vi "IR Opo Main.vi"() -> ()   [LabVIEW 2016] (continued)
        n224 = Close Reference(reference=w504, error in (no error)=w503) -> ()  [unwired: 1 out]
        n225 = Get Date/Time In Seconds() -> (seconds since 1Jan1904=w496:timestamp)
        n226 = Format Date/Time String(time format string (%c)="%m/%d/%y - %I:%M %p  ", seconds (now)=w496) -> (date/time string=w495:string)  [unwired: 1 in]
        n227 = Concatenate Strings(w495, "Camera started", "\r") -> (w500:string)
        n228 = invoke on="Log" class="Str" method="Append String"("string"=w500) -> (error out=w493:errorcluster)  [unwired: 3 in, 3 out]
        n229 = property on="Log" class="Str"(error in=w493, "Text.Scroll Position"=u32 500000) -> ()  [unwired: 1 in, 2 out]
        n230 = case shown="False" w525 {
          tunnel: [w530 w540] -> w514
          tunnel: w519 -> [w536 w540]
          tunnel: w517 -> [w535 w539]
          tunnel: [w535 w539] -> w516
          frame False {
            w528 = 1 items=["IS_DONT_WAIT", "IS_WAIT"] ("Wait")
            n231 = property class="Camera"(reference=w535, error in=w536) -> (error out=w537:errorcluster, "Acquisition"=w538:refnum<k24>)  [unwired: 1 out]
            n232 = invoke class="Acquisition" method="Capture"(reference=w538, error in=w537, "param"=w528) -> (reference out=w531:refnum<k24>, error out=w532:errorcluster, "Capture"=w529:i32)  [unwired: 1 in, 1 out]
            n233 = invoke class="Acquisition" method="ToString"(reference=w531, error in=w532) -> (error out=w534:errorcluster, "ToString"=w533:string)  [unwired: 1 in, 1 out]
            n234 = call "uc480_Error_Handling.vi"("Error Code"=w529, "Error String"=w533, "Error In"=w534) -> ("Error Out"=w530:errorcluster)  [unwired: 8 in]
          }
          frame True {
          }
        }
      }
    }
    n235 = call "uc480_SubVI_Example_SyncEventLoop.vi"("Error In"=w54, "use sync"=w56, ".NET (Reference)"=w55) -> ("Error Out"=w52:errorcluster, "Synchronize (ms)"=w53:dbl)  [unwired: 7 in]
    "Error Out" <- w52
    n236 = Wait Until Next ms Multiple(millisecond multiple=w53) -> ()  [unwired: 1 out]
  }
  n237 = flat-sequence "Initialization sequence" {
    tunnel: [w562] -> w8
    tunnel: [w546] -> w6
    tunnel: [w545] -> w5
    tunnel: [w542] -> w3
    tunnel: [w541] -> w2
    tunnel: w8 -> [w701]
    tunnel: [w695] -> w7
    tunnel: w6 -> [w694]
    tunnel: w5 -> [w693]
    tunnel: [w692] -> w4
    tunnel: w3 -> [w692]
    tunnel: w2 -> [w691]
    tunnel: [w691] -> w1
    tunnel: [w713] -> w19
    tunnel: [w704] -> w18
    tunnel: [w705] -> w14
    tunnel: w7 -> [w709]
    tunnel: w4 -> [w703]
    tunnel: w1 -> [w702]
    tunnel: w19 -> [w716]
    tunnel: [w716] -> w17
    tunnel: w18 -> [w715]
    tunnel: [w714] -> w15
    tunnel: w14 -> [w714]
    tunnel: w17 -> [w720]
    tunnel: [w720] -> w16
    tunnel: w15 -> [w719]
    tunnel: [w727] -> w13
    tunnel: w16 -> [w727]
    tunnel: w13 -> [w729]
    tunnel: [w729] -> w12
    tunnel: w12 -> [w731]
    tunnel: [w731] -> w11
    tunnel: w11 -> [w733]
    tunnel: [w733] -> w10
    tunnel: w10 -> [w735]
    tunnel: [w735] -> w9
    tunnel: w9 -> [w736]
    frame #0 {
      w563 = "standby" ("regular expression")
      w573 = FALSE ("Visible")
      n238 = control-ref of="This VI"() -> (w574:refnum<vi>)
      n239 = control-ref of="This VI"() -> (w572:refnum<vi>)
      n240 = invoke class="VI" method="Default Vals.Reinit All"(reference=w574) -> ()  [unwired: 2 in, 3 out]
      n241 = property on="Axes Manual Control" class="Bool (strict)"("Visible"=w573) -> ()  [unwired: 2 in, 2 out]
      n242 = property on="Home Axes" class="Bool"("Visible"=w573) -> ()  [unwired: 2 in, 2 out]
      n243 = property class="VI"(reference=w572) -> ("Path"=w571:path)  [unwired: 1 in, 2 out]
      n244 = Strip Path(path=w571) -> (stripped path=w570:path)  [unwired: 1 out]
      n245 = Build Path(base path=w570, name or relative path="General_Configuration.ini") -> (appended path=w568:path)
      n246 = call <vilib>:"Open Config Data.vi"("create file if necessary (T)"=FALSE, "configuration file path"=w568) -> ("error out"=w543:errorcluster, "refnum"=w544:T5)  [unwired: 7 in, 1 out]
      n247 = call "Configuration reader.vi"("refnum"=w544, "error in (no error)"=w543) -> ("Velocity"=→"Velocity":dbl, "X offset"=w555:i32, "Y travel"=w553:dbl, "X travel"=w552:dbl, "Y offset"=w554:i32, "Acceleration"=→"Acceleration":dbl, "Width (px)"=w557:i32, "Speed (µm/s)"=w561:i32, "XPS_Address"=→"XPS_Address":string, "Axis 1 group"=w542:i32, "Precision (%)"=w558:dbl, "Pixel size"=w559:dbl, "Heigth (px)"=w556:i32, "Laser Com Delay"=w545:i32, "Height  step \ndivider"=w560:i32, "VISA Laser port"=w546:string, "Axis 2 group"=w541:i32, "error out"=w548:errorcluster)
      "VISA Laser port" <- w546
      "Laser Com Delay" <- w545
      "Axis 1 group" <- w542
      "Axis 2 group" <- w541
      n248 = local write "Height  step \ndivider"(w560) -> ()
      n249 = local write "Heigth (px)"(w556) -> ()
      n250 = local write "Pixel size"(w559) -> ()
      n251 = local write "Precision (%)"(w558) -> ()
      n252 = local write "Speed (µm/s)"(w561) -> ()
      n253 = local write "Width (px)"(w557) -> ()
      n254 = local write "X offset"(w555) -> ()
      n255 = local write "X travel"(w552) -> ()
      n256 = local write "Y offset"(w554) -> ()
      n257 = local write "Y travel"(w553) -> ()
      n258 = call "CheckStatus.vi"("Error In"=w548, "delay before read (ms)"=w545, "VISA resource name"=w546) -> ("Error Out"=w547:errorcluster, "read buffer"=w566:string)  [unwired: 5 in, 2 out]
      n259 = xnode "Match Regular Expression"("input string"=w566, "regular expression"=w563, "error in"=w547) -> ("whole match"=w564:string, "error out"=w562:errorcluster)  [unwired: 3 in, 3 out]
      n260 = Equal?(x=w564, y=w563) -> (x = y?=w565:bool)
      n261 = case shown="True" w565 {
        frame False {
        }
        frame True {
          n262 = control-ref of="Log"() -> (w690:refnum<vi>)
          n263 = call "Log writer.vi"("reference"=w690, "string"="Initializing the ICE450 Ultra..." ("Initialiazation")) -> ()  [unwired: 10 in]
        }
      }
    }
    frame #1 {
      n264 = call "ICE450 Ultra Initialization.vi"("error in (no error)"=w701, "delay before read (ms)"=w693, "VISA resource name"=w694) -> ("Error Out"=w695:errorcluster, "Repetition rate"=w696:dbl, "Laser initialization status"=w700:string)  [unwired: 6 in]
      n265 = local write "Repetition\nRate (Hz)"(w696) -> ()
      n266 = property on="Log" class="Str"("Text.Scroll Position"=u32 500000) -> ()  [unwired: 2 in, 2 out]
      n267 = Concatenate Strings(w700, "\r") -> (w698:string)
      n268 = invoke on="Log" class="Str" method="Append String"("string"=w698) -> ()  [unwired: 3 in, 4 out]
    }
    frame #2 {
      n269 = local read "XPS_Address"() -> (w706:string)
      n270 = control-ref of="Log"() -> (w707:refnum<vi>)
      n271 = call "Axes initialization.vi"("Axis 2 group"=w702, "Axis 1 group"=w703, "error in (no error)"=w709, "Axis Initial Parameters"="Axis Initial Parameters", "reference"=w707, "XPS_Address"=w706) -> ("Error out"=w710:errorcluster, "Axis 1"=→"Axis 1":string, "Axis 1 ready?"=w704:bool, "Axis 2"=→"Axis 2":string, "Axes 2 ready?"=w705:bool)
      n272 = call <vilib>:"Simple Error Handler.vi"("error in (no error)"=w710) -> ()  [unwired: 4 in, 5 out]
      n273 = And(x=w704, y=w705) -> (x .and. y?=w713:bool)
    }
    frame #3 {
      n274 = case shown="True" w715 {
        frame False {
        }
        frame True {
          n275 = control-ref of="Log"() -> (w718:refnum<vi>)
          n276 = call "Log writer.vi"("reference"=w718, "string"="Axis 1 ready" ("Initialiazation")) -> ()  [unwired: 10 in]
        }
      }
    }
    frame #4 {
      n277 = case shown="True" w719 {
        frame False {
        }
        frame True {
          n278 = control-ref of="Log"() -> (w721:refnum<vi>)
          n279 = call "Log writer.vi"("reference"=w721, "string"="Axis 2 ready" ("Initialiazation")) -> ()  [unwired: 10 in]
        }
      }
    }
    frame #5 {
      w723 = FALSE ("Visible")
      # "Set defaults"
      n280 = property on="LAMP" class="Bool (strict)"("BoolText.Text"="LAMP OFF" ("Boolean Text.Text")) -> ()  [unwired: 2 in, 2 out]
      n281 = property on="Laser Operation" class="Bool (strict)"("Blinking"=w723) -> ()  [unwired: 2 in, 2 out]
      n282 = property on="Capture" class="Bool"("Visible"=w723) -> ()  [unwired: 2 in, 2 out]
      n283 = property on="SINGLE SHOT" class="Bool"("Visible"=w723) -> ()  [unwired: 2 in, 2 out]
      n284 = property on="LASER" class="Bool (strict)"("BoolText.Text"="LASER OFF" ("Boolean Text.Text"), "Visible"=FALSE) -> ()  [unwired: 2 in, 2 out]
    }
    frame #6 {
      n285 = local write "Camera Status"("Init camera" ("Camera Status")) -> ()
    }
    frame #7 {
      n286 = Wait (ms)(milliseconds to wait=u32 1000) -> ()  [unwired: 1 out]
    }
    frame #8 {
      n287 = local write "Camera Status"("Start live") -> ()
    }
    frame #9 {
      n288 = Wait (ms)(milliseconds to wait=u32 1000) -> ()  [unwired: 1 out]
    }
    frame #10 {
      n289 = case shown="True" w736 {
        frame False {
          n290 = One Button Dialog(message="Axes not ready") -> ()  [unwired: 1 in, 1 out]
        }
        frame True {
          n291 = property on="Axes Manual Control" class="Bool (strict)"("Visible"=TRUE) -> ()  [unwired: 2 in, 2 out]
          n292 = property on="Home Axes" class="Bool"("Visible"=TRUE) -> ()  [unwired: 2 in, 2 out]
          n293 = control-ref of="Log"() -> (w739:refnum<vi>)
          n294 = call "Log writer.vi"("reference"=w739, "string"="System ready" ("Initialiazation")) -> ()  [unwired: 10 in]
        }
      }
    }
  }
  n295 = while "Laser control & Stages Control" {
    stop <- w754 stop-if-true
    n296 = local read "Laser Com Delay"() -> (w742:i32)
    n297 = local read "VISA Laser port"() -> (w743:string)
    n298 = local read "XPS_Address"() -> (w746:string)
    n299 = local read "Axis 2"() -> (w744:string)
    n300 = local read "Axis 1"() -> (w745:string)
    n301 = event shown="[11] \"Process Image\": Value Change" {
      selector: _ -> [_ _ _ _ _ _ _ _ _ _ _ _ _ _ _ _ _ _ _ _]
      dyn-events: _ -> [_ _ _ _ _ _ _ _ _ _ _ _ _ _ _ _ _ _ _ _]
      timeout: _ -> [_ _ _ _ _ _ _ _ _ _ _ _ _ _ _ _ _ _ _ _]
      tunnel: [_ _ _ w1086 _ _ _ _ _ _ _ _ _ _ _ _ _ _ _ _] -> w754
      tunnel: [w761 w917 w1080 _ _ _ w1141 _ w1169 w1196 _ w1257 _ _ _ "" ("StringOut") w1516 _ w1640 w1743] -> w747
      tunnel: w746 -> [_ _ _ _ _ _ _ _ _ w1199 _ _ _ _ _ w1435 w1515 _ w1627 w1732]
      tunnel: w745 -> [_ _ _ _ _ _ _ _ _ w1198 _ _ _ _ _ w1434 w1514 _ w1626 w1744]
      tunnel: w744 -> [_ _ _ _ _ _ _ _ _ w1197 _ _ _ _ _ w1433 w1513 _ w1625 w1745]
      tunnel: w743 -> [w759 w915 w1077 w1085 _ _ w1144 w1164 _ _ _ _ _ _ _ _ _ _ _ _]
      tunnel: w742 -> [w758 w914 w1076 w1084 _ _ w1143 w1163 _ _ _ _ _ _ _ _ _ _ _ _]
      event "LAMP": Value Change {
        n302 = event-data() -> ()  [unwired: 1 in, 6 out]
        n303 = case shown="True" "LAMP" {
          tunnel: [w762 w890] -> w761
          tunnel: w759 -> [w768 w889]
          tunnel: w758 -> [w767 w888]
          frame False {
            w763 = "standby" ("regular expression")
            n304 = call "FLStop.vi"("delay before read (ms)"=w767, "VISA resource name"=w768) -> ("read buffer"=w766:string)  [unwired: 6 in, 3 out]
            n305 = xnode "Match Regular Expression"("input string"=w766, "regular expression"=w763) -> ("whole match"=w764:string)  [unwired: 4 in, 4 out]
            n306 = Equal?(x=w764, y=w763) -> (x = y?=w765:bool)
            n307 = case shown="True" w765 {
              tunnel: ["" "Flashlamp deactivated"] -> w762
              frame False {
              }
              frame True {
                w770 = FALSE ("Visible")
                n308 = property on="LASER" class="Bool (strict)"("Visible"=w770) -> ()  [unwired: 2 in, 2 out]
                n309 = property on="Capture" class="Bool"("Visible"=w770) -> ()  [unwired: 2 in, 2 out]
                n310 = property on="SINGLE SHOT" class="Bool"("Visible"=w770) -> ()  [unwired: 2 in, 2 out]
                n311 = property on="Laser Operation" class="Bool (strict)"("Blinking"=w770) -> ()  [unwired: 2 in, 2 out]
                n312 = property on="LAMP" class="Bool (strict)"("BoolText.Text"="LAMP OFF" ("Boolean Text.Text")) -> ()  [unwired: 2 in, 2 out]
              }
            }
          }
          frame True {
            n313 = flat-sequence {
              tunnel: w889 -> [w898]
              tunnel: w888 -> [w897]
              tunnel: [w894] -> w887
              tunnel: [w908] -> w890
              tunnel: w887 -> [w907]
              frame #0 {
                w895 = "fire" ("regular expression")
                n314 = while {
                  i -> [w902]
                  stop <- w905 stop-if-true
                  n315 = Wait Until Next ms Multiple(millisecond multiple=u32 1000) -> ()  [unwired: 1 out]
                  n316 = Equal?(x=5, y=w902) -> (x = y?=w905:bool)
                  n317 = Subtract(x=5, y=w902) -> (x-y=w900:i32)
                  n318 = Number To Decimal String(number=w900) -> (decimal integer string=w901:string)  [unwired: 1 in]
                  n319 = property on="LAMP" class="Bool (strict)"("BoolText.Text"=w901) -> ()  [unwired: 2 in, 2 out]
                }
                n320 = Wait (ms)(milliseconds to wait=u32 5000) -> ()  [unwired: 1 out]
                n321 = call "FLStart.vi"("delay before read (ms)"=w897, "VISA resource name"=w898) -> ("Error Out"=w892:errorcluster, "read buffer"=w893:string)  [unwired: 6 in, 2 out]
                n322 = Match Pattern(string=w893, regular expression=w895) -> (match substring=w896:string)  [unwired: 1 in, 3 out]
                n323 = call <vilib>:"Simple Error Handler.vi"("error source (\" \")"="Lamp" ("error source (\" \")"), "error in (no error)"=w892) -> ()  [unwired: 3 in, 5 out]
                n324 = Equal?(x=w896, y=w895) -> (x = y?=w894:bool)
              }
              frame #1 {
                n325 = case shown="True" w907 {
                  tunnel: ["Flashlamp NOT firing" "Flashlamp activated"] -> w908
                  frame False {
                    n326 = property on="LAMP" class="Bool (strict)"("Value"=FALSE ("LAMP")) -> ()  [unwired: 2 in, 2 out]
                  }
                  frame True {
                    w911 = TRUE ("Visible")
                    n327 = property on="LASER" class="Bool (strict)"("Visible"=w911) -> ()  [unwired: 2 in, 2 out]
                    n328 = property on="Capture" class="Bool"("Visible"=w911) -> ()  [unwired: 2 in, 2 out]
                    n329 = property on="LAMP" class="Bool (strict)"("BoolText.Text"="LAMP ON" ("Boolean Text.Text")) -> ()  [unwired: 2 in, 2 out]
                    n330 = property on="SINGLE SHOT" class="Bool"("Visible"=w911) -> ()  [unwired: 2 in, 2 out]
                  }
                }
              }
            }
          }
        }
      }
      event "LASER": Value Change {
        n331 = event-data() -> ()  [unwired: 1 in, 6 out]
        n332 = case shown="False" "LASER" {
          tunnel: [w928 w1057] -> w918
          tunnel: [w927 w1056] -> w917
          tunnel: w915 -> [w925 w1051]
          tunnel: w914 -> [w924 w1050]
          frame False {
            w922 = "fire" ("regular expression")
            n333 = local read "LAMP"() -> (w926:bool)
            n334 = case shown="True" w926 {
              tunnel: [FALSE ("Visible") TRUE ("Visible")] -> w919
              frame False {
              }
              frame True {
              }
            }
            n335 = property on="Capture" class="Bool"("Visible"=w919) -> ()  [unwired: 2 in, 2 out]
            n336 = property on="SINGLE SHOT" class="Bool"("Visible"=w919) -> ()  [unwired: 2 in, 2 out]
            n337 = call "QSStop.vi"("delay before read (ms)"=w924, "VISA resource name"=w925) -> ("read buffer"=w921:string)  [unwired: 6 in, 3 out]
            n338 = xnode "Match Regular Expression"("input string"=w921, "regular expression"=w922) -> ("whole match"=w923:string)  [unwired: 4 in, 4 out]
            n339 = Equal?(x=w923, y=w922) -> (x = y?=w920:bool)
            n340 = case shown="False" w920 {
              tunnel: [FALSE w932] -> w928
              tunnel: ["" "Q-Switch deactivated"] -> w927
              frame False {
              }
              frame True {
                w932 = FALSE ("Boolean")
                n341 = property on="LASER" class="Bool (strict)"("BoolText.Text"="LASER OFF" ("Boolean Text.Text"), "Value"=w932) -> ()  [unwired: 2 in, 2 out]
                n342 = property on="Laser Operation" class="Bool (strict)"("Blinking"=w932) -> ()  [unwired: 2 in, 2 out]
              }
            }
          }
          frame True {
            w1053 = "fire" ("regular expression")
            n343 = call "CheckStatus.vi"("delay before read (ms)"=w1050, "VISA resource name"=w1051) -> ("read buffer"=w1055:string)  [unwired: 6 in, 3 out]
            n344 = Match Pattern(string=w1055, regular expression=w1053) -> (match substring=w1054:string)  [unwired: 1 in, 3 out]
            n345 = Equal?(x=w1054, y=w1053) -> (x = y?=w1052:bool)
            n346 = case shown="True" w1052 {
              tunnel: [FALSE ("Boolean") w1068] -> w1057
              tunnel: ["The flashlamp is not firing" w1067] -> w1056
              tunnel: w1051 -> [_ w1066]
              tunnel: w1050 -> [_ w1065]
              frame False {
                n347 = property on="LASER" class="Bool (strict)"("Value"=FALSE ("LASER")) -> ()  [unwired: 2 in, 2 out]
              }
              frame True {
                w1063 = "qs" ("regular expression")
                n348 = call "QSStart.vi"("delay before read (ms)"=w1065, "VISA resource name"=w1066) -> ("read buffer"=w1062:string)  [unwired: 6 in, 3 out]
                n349 = Match Pattern(string=w1062, regular expression=w1063) -> (match substring=w1064:string)  [unwired: 1 in, 3 out]
                n350 = Equal?(x=w1064, y=w1063) -> (x = y?=w1061:bool)
                n351 = case shown="True" w1061 {
                  tunnel: [FALSE ("Boolean") w1074] -> w1068
                  tunnel: ["Q-Switch is NOT firing" "Q-Switch activated"] -> w1067
                  frame False {
                    n352 = property on="LASER" class="Bool (strict)"("Value"=FALSE ("LASER")) -> ()  [unwired: 2 in, 2 out]
                  }
                  frame True {
                    w1072 = FALSE ("Visible")
                    w1074 = TRUE ("Boolean")
                    n353 = property on="Capture" class="Bool"("Visible"=w1072) -> ()  [unwired: 2 in, 2 out]
                    n354 = property on="Laser Operation" class="Bool (strict)"("Blinking"=w1074) -> ()  [unwired: 2 in, 2 out]
                    n355 = property on="LASER" class="Bool (strict)"("BoolText.Text"="LASER ON" ("Boolean Text.Text")) -> ()  [unwired: 2 in, 2 out]
                    n356 = property on="SINGLE SHOT" class="Bool"("Visible"=w1072) -> ()  [unwired: 2 in, 2 out]
                  }
                }
              }
            }
          }
        }
        "Laser Operation" <- w918
      }
      event "Repetition\nRate (Hz)": Value Change {
        n357 = event-data() -> ()  [unwired: 1 in, 6 out]
        n358 = call "FLFrequencySet.vi"("Frequency (Hz)"="Repetition\nRate (Hz)", "delay before read (ms)"=w1076, "VISA resource name"=w1077) -> ()  [unwired: 5 in, 4 out]
        n359 = Number To Fractional String(number="Repetition\nRate (Hz)", precision (6)=i16 2 ("width (-)")) -> (F-format string=w1082:string)  [unwired: 2 in]
        n360 = Concatenate Strings("Repetition rate set to: " ("string"), w1082, " Hz" ("string")) -> (w1080:string)
      }
      event "EXIT": Value Change {
        n361 = event-data() -> ()  [unwired: 1 in, 6 out]
        n362 = flat-sequence {
          tunnel: w1085 -> [w1088]
          tunnel: w1084 -> [w1087]
          tunnel: ["EXIT"] -> w1086
          frame #0 {
            n363 = call "QSStop.vi"("delay before read (ms)"=w1087, "VISA resource name"=w1088) -> ("Error Out"=w1089:errorcluster)  [unwired: 6 in, 3 out]
            n364 = call "FLStop.vi"("Error In"=w1089, "delay before read (ms)"=w1087, "VISA resource name"=w1088) -> ()  [unwired: 5 in, 4 out]
          }
          frame #1 {
            n365 = Wait (ms)(milliseconds to wait=u32 1000) -> ()  [unwired: 1 out]
          }
          frame #2 {
            n366 = local write "Camera Status"("Exit camera") -> ()
          }
          frame #3 {
            n367 = Wait (ms)(milliseconds to wait=u32 1000) -> ()  [unwired: 1 out]
          }
          frame #4 {
            n368 = control-ref of="This Application"() -> (w1112:refnum<vi>)
            n369 = control-ref of="This VI"() -> (w1096:refnum<vi>)
            n370 = property class="VI"(reference=w1096) -> ("Path"=w1097:path)  [unwired: 1 in, 2 out]
            n371 = property class="App"(reference=w1112) -> ("App.Kind"=w1111:T8)  [unwired: 1 in, 2 out]
            n372 = Strip Path(path=w1097) -> (stripped path=w1106:path)  [unwired: 1 out]
            n373 = case shown="\"Run Time System\"" w1111 {
              frame "Development System", Default {
              }
              frame "Run Time System" {
                n374 = control-ref of="This VI"() -> (w1121:refnum<vi>)
                n375 = invoke class="VI" method="FP.Close"(reference=w1121) -> ()  [unwired: 2 in, 3 out]
                n376 = Quit LabVIEW() -> ()  [unwired: 1 in]
              }
            }
            n377 = Build Path(base path=w1106, name or relative path="Logs") -> (appended path=w1104:path)
            n378 = call <vilib>:"Check if File or Folder Exists.vi"("path"=w1104) -> ("file or folder exists?"=w1105:bool, "dup path"=w1107:path)  [unwired: 8 in, 1 out]
            n379 = case shown="False" w1105 {
              tunnel: w1107 -> [w1114 w1115]
              tunnel: [w1113 w1115] -> w1110
              frame False {
                n380 = Create Folder(path (use dialog)=w1114) -> (created path=w1113:path)  [unwired: 2 in, 2 out]
              }
              frame True {
              }
            }
            n381 = Get Date/Time In Seconds() -> (seconds since 1Jan1904=w1101:timestamp)
            n382 = Format Date/Time String(time format string (%c)="%d%m%y %I-%M %p ", seconds (now)=w1101) -> (date/time string=w1099:string)  [unwired: 1 in]
            n383 = Concatenate Strings(w1099, "Log File.txt") -> (w1109:string)
            n384 = Build Path(base path=w1110, name or relative path=w1109) -> (appended path=w1108:path)
            n385 = Open/Create/Replace File(file path (use dialog)=w1108, operation (0:open)=T6."replace or create") -> (refnum out=w1095:refnum<file>, cancelled=w1093:bool, error out=w1094:errorcluster)  [unwired: 4 in]
            n386 = case shown="False" w1093 {
              tunnel: w1095 -> [w1120 _]
              tunnel: w1094 -> [w1118 _]
              frame False {
                n387 = local read "Log"() -> (w1119:string)
                n388 = Write to Text File(file (use dialog)=w1120, text=w1119, error in=w1118) -> (refnum out=w1117:refnum<file>, error out=w1116:errorcluster)  [unwired: 2 out]
                n389 = Close File(refnum=w1117, error in=w1116) -> ()  [unwired: 2 out]
              }
              frame True {
              }
            }
          }
          frame #5 {
          }
        }
      }
      event "Processing time unit", "Processi time (sec)": Value Change {
        n390 = event-data() -> ()  [unwired: 1 in, 6 out]
        n391 = local read "Processing time unit"() -> (w1125:string)
        n392 = Equal?(x=w1125, y="min") -> (x = y?=w1123:bool)
        n393 = case shown="False" w1123 {
          frame False {
            n394 = local read "Processi time (sec)"() -> (w1126:i32)
            n395 = local write "Process time"(w1126) -> ()
          }
          frame True {
            n396 = local read "Processi time (sec)"() -> (w1128:i32)
            n397 = Quotient & Remainder(x=w1128, y=60) -> (floor(x/y)=w1127:i32)  [unwired: 1 out]
            n398 = local write "Process time"(w1127) -> ()
          }
        }
      }
      event "Overlay MSI Image": Value Change {
        n399 = event-data() -> ()  [unwired: 1 in, 6 out]
        n400 = vi-ref "MSI_Image_overlap.vi"() -> (w1130:refnum<vi>)
        n401 = case shown="True" "Overlay MSI Image" {
          tunnel: w1130 -> [_ w1135]
          frame False {
          }
          frame True {
            n402 = invoke class="VI" method="FP.Open"(reference=w1135, "Activate"=TRUE ("Activate?"), "State"=T7."Standard") -> (reference out=w1138:refnum<vi>, error out=w1133:errorcluster)  [unwired: 2 in, 3 out]
            n403 = invoke class="VI" method="Run VI"(reference=w1138, error in=w1133, "Wait until done"=FALSE ("Wait Until Done"), "Auto Dispose Ref"=TRUE ("Auto Dispose Reference")) -> (reference out=w1134:refnum<vi>, error out=w1132:errorcluster)  [unwired: 1 in, 3 out]
            n404 = Close Reference(reference=w1134, error in (no error)=w1132) -> ()  [unwired: 1 out]
          }
        }
      }
      event "SINGLE SHOT": Value Change {
        n405 = event-data() -> ()  [unwired: 1 in, 6 out]
        n406 = case shown="True" "SINGLE SHOT" {
          tunnel: w1144 -> [_ w1148]
          tunnel: w1143 -> [_ w1147]
          tunnel: ["" w1146] -> w1141
          frame False {
          }
          frame True {
            w1152 = "fire" ("regular expression")
            n407 = call "CheckStatus.vi"("delay before read (ms)"=w1147, "VISA resource name"=w1148) -> ("read buffer"=w1150:string)  [unwired: 6 in, 3 out]
            n408 = Match Pattern(string=w1150, regular expression=w1152) -> (match substring=w1151:string)  [unwired: 1 in, 3 out]
            n409 = Equal?(x=w1151, y=w1152) -> (x = y?=w1149:bool)
            n410 = case shown="True" w1149 {
              tunnel: ["The flashlamp is not firing" w1160] -> w1146
              tunnel: w1148 -> [_ w1159]
              tunnel: w1147 -> [_ w1158]
              frame False {
              }
              frame True {
                w1156 = "qs" ("regular expression")
                n411 = call "QSSingleShot.vi"("delay before read (ms)"=w1158, "VISA resource name"=w1159) -> ("read buffer"=w1155:string)  [unwired: 6 in, 3 out]
                n412 = Match Pattern(string=w1155, regular expression=w1156) -> (match substring=w1157:string)  [unwired: 1 in, 3 out]
                n413 = Equal?(x=w1157, y=w1156) -> (x = y?=w1154:bool)
                n414 = case shown="True" w1154 {
                  tunnel: ["Q-Switch is NOT firing" "Q-Switch activated"] -> w1160
                  frame False {
                  }
                  frame True {
                  }
                }
              }
            }
          }
        }
      }
      event "Laser Status": Value Change {
        n415 = event-data() -> ()  [unwired: 1 in, 6 out]
        n416 = case shown="True" "Laser Status" {
          tunnel: w1164 -> [_ w1167]
          tunnel: w1163 -> [_ w1166]
          frame False {
          }
          frame True {
            n417 = call "ICE450UltraMonitor.vi"("delay before read (ms)"=w1166, "VISA resource name"=w1167) -> ()  [unwired: 10 in]
          }
        }
      }
      event "Open \nManual": Value Change {
        n418 = event-data() -> ()  [unwired: 1 in, 6 out]
        n419 = case shown="True" "Open \nManual" {
          tunnel: [_ "Opening Manual" ("StringOut")] -> w1169
          frame False {
          }
          frame True {
            w1178 = FALSE  # wait until completion? (T)
            n420 = control-ref of="This VI"() -> (w1182:refnum<vi>)
            n421 = property class="VI"(reference=w1182) -> ("Path"=w1181:path)  [unwired: 1 in, 2 out]
            n422 = Strip Path(path=w1181) -> (stripped path=w1180:path)  [unwired: 1 out]
            n423 = Build Path(base path=w1180, name or relative path="LAST_Software_Manual.PDF") -> (appended path=w1172:path)
            n424 = Path To String(path=w1172) -> (string=w1175:string)
            n425 = Concatenate Strings("cmd  /c \"", w1175, "\"" ("string")) -> (w1170:string)
            n426 = call <vilib>:"System Exec.vi"("run minimized? (F)"=TRUE, "wait until completion? (T)"=w1178, "error in (no error)"="error in (no error)", "command line"=w1170) -> ("error out"=→"error out":errorcluster)  [unwired: 4 in, 3 out]
          }
        }
      }
      event "Stages status": Value Change {
        w1190 = "Ready"
        n427 = event-data() -> ()  [unwired: 1 in, 6 out]
        n428 = case shown="True" "Stages status" {
          tunnel: w1199 -> [_ w1212]
          tunnel: w1198 -> [_ w1211]
          tunnel: w1197 -> [_ w1210]
          tunnel: [w1203 w1209] -> w1196
          tunnel: [w1203 w1207] -> w1186
          tunnel: [w1203 w1208] -> w1185
          frame False {
            w1203 = ""
          }
          frame True {
            n429 = call <userlib>:"Open TCP-IP.vi"("IP address"=w1212) -> ("error out"=w1206:errorcluster, "Connection ID"=w1213:T9)  [unwired: 8 in, 1 out]
            n430 = call <vilib>:"Simple Error Handler.vi"("error in (no error)"=w1206) -> ("error?"=w1204:bool, "error out"=w1205:errorcluster)  [unwired: 4 in, 3 out]
            n431 = case shown="False" w1204 {
              tunnel: w1213 -> [w1234 _]
              tunnel: w1205 -> [w1233 _]
              tunnel: w1211 -> [w1226 _]
              tunnel: w1210 -> [w1225 _]
              tunnel: [w1224 w1235] -> w1209
              tunnel: [w1221 w1235] -> w1208
              tunnel: [w1217 w1235] -> w1207
              frame False {
                n432 = call "Get Stages Status.vi"("error in (no error)"=w1233, "Group Name (250 c max)"=w1226, "connection ID in"=w1234) -> ("error out"=w1230:errorcluster, "XPS error out"=w1229:errorcluster, "Group Status String"=w1221:string, "connection ID out"=w1232:T9)  [unwired: 4 in, 1 out]
                n433 = call "Get Stages Status.vi"("error in (no error)"=w1230, "XPS error in (no error)"=w1229, "Group Name (250 c max)"=w1225, "connection ID in"=w1232) -> ("error out"=w1227:errorcluster, "XPS error out"=w1223:errorcluster, "Group Status String"=w1217:string, "connection ID out"=w1228:T9)  [unwired: 3 in, 1 out]
                n434 = call <vilib>:"Simple Error Handler.vi"("error source (\" \")"="Stage status" ("error source (\" \")"), "error in (no error)"=w1223) -> ()  [unwired: 3 in, 5 out]
                n435 = Concatenate Strings("Axis 1 " ("string"), w1221) -> (w1220:string)
                n436 = call <userlib>:"Close TCP-IP.vi"("error in (no error)"=w1227, "connection ID in"=w1228) -> ("Error out"=w1222:errorcluster)  [unwired: 9 in]
                n437 = call <vilib>:"Simple Error Handler.vi"("error source (\" \")"="TCP close Stage status" ("error source (\" \")"), "error in (no error)"=w1222) -> ()  [unwired: 3 in, 5 out]
                n438 = Concatenate Strings("Axis 2 " ("string"), w1217) -> (w1218:string)
                n439 = Concatenate Strings(w1220, " - " ("string"), w1218) -> (w1224:string)
              }
              frame True {
                w1235 = ""
              }
            }
          }
        }
        n440 = String Subset(string=w1185, offset (0)=0, length (rest)=5 ("length (rest)")) -> (substring=w1189:string)
        n441 = String Subset(string=w1186, offset (0)=0, length (rest)=5 ("length (rest)")) -> (substring=w1191:string)
        n442 = Equal?(x=w1190, y=w1189) -> (x = y?=w1187:bool)
        n443 = Equal?(x=w1191, y=w1190) -> (x = y?=w1188:bool)
        n444 = And(x=w1188, y=w1187) -> (x .and. y?=w1184:bool)
        n445 = case shown="True" w1184 {
          frame False {
          }
          frame True {
            n446 = property on="Axes Manual Control" class="Bool (strict)"("Visible"=TRUE) -> ()  [unwired: 2 in, 2 out]
            n447 = property on="Home Axes" class="Bool"("Visible"=TRUE) -> ()  [unwired: 2 in, 2 out]
          }
        }
      }
      event "Save configuration": Value Change {
        n448 = event-data() -> ()  [unwired: 1 in, 6 out]
        n449 = case shown="True" "Save configuration" {
          frame False {
          }
          frame True {
            n450 = control-ref of="This VI"() -> (w1255:refnum<vi>)
            n451 = property class="VI"(reference=w1255) -> ("Path"=w1254:path)  [unwired: 1 in, 2 out]
            n452 = Strip Path(path=w1254) -> (stripped path=w1253:path)  [unwired: 1 out]
            n453 = local read "Height  step \ndivider"() -> (w1248:i32)
            n454 = Build Path(base path=w1253, name or relative path="General_Configuration.ini") -> (appended path=w1251:path)
            n455 = local read "Speed (µm/s)"() -> (w1244:i32)
            n456 = local read "Precision (%)"() -> (w1245:dbl)
            n457 = local read "Heigth (px)"() -> (w1247:i32)
            n458 = local read "Width (px)"() -> (w1243:i32)
            n459 = local read "Pixel size"() -> (w1246:dbl)
            n460 = local read "X offset"() -> (w1242:i32)
            n461 = local read "X travel"() -> (w1240:dbl)
            n462 = local read "Y offset"() -> (w1241:i32)
            n463 = local read "Y travel"() -> (w1239:dbl)
            n464 = call <vilib>:"Open Config Data.vi"("create file if necessary (T)"=FALSE, "configuration file path"=w1251) -> ("error out"=w1238:errorcluster, "refnum"=w1249:T5)  [unwired: 7 in, 1 out]
            n465 = call "Configuration writer.vi"("Path"=w1249, "Width (px)"=w1243, "error in (no error)"=w1238, "Precision (%)"=w1245, "Heigth (px)"=w1247, "X offset"=w1242, "X travel"=w1240, "Y offset"=w1241, "Speed (µm/s)"=w1244, "Height  step \ndivider"=w1248, "Y travel"=w1239, "Pixel size"=w1246) -> ("error out"=w1237:errorcluster)  [unwired: 7 in]
            n466 = call <vilib>:"Simple Error Handler.vi"("error in (no error)"=w1237) -> ()  [unwired: 4 in, 5 out]
          }
        }
      }
      event "Process Image": Value Change {
        n467 = event-data() -> ()  [unwired: 1 in, 6 out]
        n468 = case shown="True" "Process Image" {
          tunnel: ["" "Processing done"] -> w1257
          frame False {
          }
          frame True {
            (unwired) "untitled" ("Image Name")
            w1291 = 2 ("y")
            w1318 = 0.5  # Delay after laser on/off
            w1352 = T10 0 items=["Grayscale (U8)", "Grayscale (I16)", "Grayscale (SGL)", "Complex (CSG)", "RGB (U32)", "HSL (U32)", "RGB (U64)", "Grayscale (U16)"] ("Image Type")
            w1355 = i16 4 ("precision (6)")
            w1349 = 1000 ("y")
            n469 = control-ref of="This VI"() -> (w1263:refnum<vi>)
            n470 = control-ref of="This VI"() -> (w1271:refnum<vi>)
            n471 = local read "Source"() -> (w1354:T2)
            n472 = call "IMAQ Create"("Image Name"="untitled") -> ("New Image"=w1260:T2)  [unwired: 4 in, 1 out]
            n473 = property class="VI"(reference=w1263) -> ("Path"=w1264:path)  [unwired: 1 in, 2 out]
            n474 = property class="VI"(reference=w1271) -> ("Path"=w1270:path)  [unwired: 1 in, 2 out]
            n475 = property on="Source" class="ImageControl"() -> ("ROI"=w1261:T11)  [unwired: 2 in, 2 out]
            n476 = call "IMAQ ROIToMask 2"("ROI Descriptor"=w1261, "Image"=w1260) -> ("Image Out"=w1259:T2)  [unwired: 7 in, 2 out]
            n477 = call "IMAQ Cast Image"("Image Type"=w1352, "Image Src"=w1354) -> ("error out"=w1303:errorcluster, "Image Dst Out"=w1353:T2)  [unwired: 8 in]
            n478 = Unbundle By Name(w1261) -> ("Global Rectangle"=w1308:i32[])
            n479 = Strip Path(path=w1264) -> (stripped path=w1265:path)  [unwired: 1 out]
            n480 = Strip Path(path=w1270) -> (stripped path=w1269:path)  [unwired: 1 out]
            n481 = call "IMAQ ROIToMask 2"("error in (no error)"=w1303, "ROI Descriptor"=w1261, "Image"=w1353) -> ("error out"=w1304:errorcluster, "Image Out"=w1356:T2)  [unwired: 6 in, 1 out]
            n482 = Build Path(base path=w1265, name or relative path="Last_ROI.TIFF") -> (appended path=w1267:path)
            n483 = call-poly "IMAQ Write File 2"("File Path"=w1267, "Image"=w1259) -> ()  [unwired: 8 in, 2 out]
            n484 = Build Path(base path=w1269, name or relative path="Last_ROI.TIFF") -> ()  [unwired: 1 out]
            n485 = call "IMAQ ImageToArray"("error in (no error)"=w1304, "Image"=w1356) -> ("error out"=w1302:errorcluster, "Image Pixels (U8)"=w1274:u8[][])  [unwired: 2 in, 3 out]
            n486 = Array To Cluster(array=w1308) -> (cluster=w1307:T12)
            n487 = local read "Y offset"() -> (w1283:i32)
            n488 = local read "X offset"() -> (w1284:i32)
            n489 = call <vilib>:"Simple Error Handler.vi"("error in (no error)"=w1302) -> ()  [unwired: 4 in, 5 out]
            n490 = Unbundle(w1307) -> ("Global Rectangle[0]"=w1306:i32, "Global Rectangle[1]"=w1305:i32)
            n491 = Subtract(x=w1306, y=w1283) -> (x-y=w1297:i32)
            n492 = Subtract(x=w1305, y=w1284) -> (x-y=w1288:i32)
            n493 = local read "Width (px)"() -> (w1272:i32)
            n494 = call "ROI corrector.vi"("ROI"=w1274, "Spot diameter"=w1272) -> ("Corrected ROI"=w1273:u8[][])  [unwired: 9 in]
            n495 = Empty Array?(array=w1273) -> (empty?=w1340:bool)
            n496 = case shown="False" w1340 {
              tunnel: [w1363 u8[][] [[1]] ("Image Pixels (U8)")] -> w1339
              tunnel: w1273 -> [w1363 _]
              frame False {
              }
              frame True {
                n497 = One Button Dialog(message="ATTENTION: you did not select\nany region of interest") -> ()  [unwired: 1 in, 1 out]
              }
            }
            n498 = local read "Heigth (px)"() -> (w1290:i32)
            n499 = Divide(x=w1272, y=2.0) -> (x/y=w1279:dbl)
            n500 = Divide "Spot height radius"(x=w1290, y=w1291) -> (x/y=w1292:dbl)
            n501 = Divide "Spot width radius"(x=w1272, y=w1291) -> (x/y=w1295:dbl)
            n502 = Initialize Array(1 ("element"), w1272, w1272) -> (w1280:i32[][])
            n503 = Round To Nearest(number=w1279) -> (nearest integer value=w1277:dbl)
            n504 = call "circle spot calculator.vi"("Center Y"=w1277, "Radius"=w1277, "Center X"=w1277, "initialized array"=w1280) -> ("Array"=w1276:i32[][])  [unwired: 6 in]
            n505 = Round To Nearest(number=w1292) -> (nearest integer value=w1289:dbl)
            n506 = Round To Nearest(number=w1295) -> (nearest integer value=w1294:dbl)
            n507 = local read "Pixel size"() -> (w1285:dbl)
            n508 = Add Array Elements(numeric array=w1276) -> (sum=w1275:i32)
            n509 = Add(x=w1289, y=w1288) -> (x+y=w1287:dbl)
            n510 = Add(x=w1294, y=w1297) -> (x+y=w1296:dbl)
            n511 = Multiply(x=w1287, y=w1285) -> (x*y=w1286:dbl)
            n512 = Multiply(x=w1285, y=w1296) -> (x*y=w1293:dbl)
            n513 = Multiply(x=w1285, y=w1285) -> (x*y=w1343:dbl)
            n514 = To Double Precision Float(number=w1339) -> (double precision float=w1341:dbl[][])
            n515 = Array Size(array=w1339) -> (size(s)=w1357:i32[])
            n516 = local read "Height  step \ndivider"() -> (w1300:i32)
            n517 = Divide(x=w1293, y=w1349) -> (x/y=w1351:dbl)
            n518 = Divide(x=w1286, y=w1349) -> (x/y=w1350:dbl)
            n519 = Add Array Elements(numeric array=w1341) -> (sum=w1345:dbl)
            n520 = Array To Cluster(array=w1357) -> (cluster=w1358:cluster{"[0]":i32, "[1]":i32})
            n521 = Number To Fractional String(number=w1351, precision (6)=w1355) -> (F-format string=w1337:string)  [unwired: 2 in]
            n522 = Number To Fractional String(number=w1350, precision (6)=w1355) -> (F-format string=w1338:string)  [unwired: 2 in]
            n523 = Unbundle(w1358) -> ("[0]"=w1301:i32, "[1]"=w1312:i32)
            n524 = Divide(x=w1345, y=u8 255) -> (x/y=w1342:dbl)
            n525 = Multiply(x=w1342, y=w1343) -> (x*y=w1334:dbl)
            n526 = Multiply(x=w1301, y=w1285) -> (x*y=w1330:dbl)
            n527 = Multiply(x=w1312, y=w1285) -> (x*y=w1331:dbl)
            n528 = Fract/Exp String To Number(string=w1337) -> (number=→"Axis 1 Offset":dbl)  [unwired: 3 in, 1 out]
            n529 = Fract/Exp String To Number(string=w1338) -> (number=→"Axis 2 Offset":dbl)  [unwired: 3 in, 1 out]
            n530 = Divide "Height of a line"(x=w1290, y=w1300) -> (x/y=w1310:dbl)
            n531 = Multiply(x=w1285, y=w1310) -> (x*y=w1311:dbl)
            n532 = Round To Nearest(number=w1330) -> (nearest integer value=→"ROI container\nheigth (µm)":dbl)
            n533 = Round To Nearest(number=w1331) -> (nearest integer value=→"ROI container\nwidth (µm)":dbl)
            n534 = Divide(x=w1334, y=1000000.0) -> (x/y=→"ROI Area \n(mm2)":dbl)
            n535 = call "ROI parser.vi"("Circle spot"=w1275, "Circle?"="Circle?", "ROI (8 bit image)"=w1339, "Ablation spot width"=w1272, "Sampling\nPrecision"=w1300, "Ablation spot heigth"="Precision (%)", "Height  step \ndivider"=w1290) -> ("Parsed array"=w1362:bool[][])  [unwired: 4 in]
            n536 = call "Array processor.vi"("Source array"=w1362, "Pixel size"=w1285) -> ("Lenght array"=w1298:dbl[][], "T/F product array"=w1325:bool[][])  [unwired: 8 in]
            n537 = Array Size(array=w1325) -> (size(s)=w1324:i32[])
            n538 = Index Array(array=w1325, index (col)=0 ("disabled index (col)")) -> (element=w1360:bool[])  [unwired: 1 in]
            n539 = Array Size(array=w1360) -> (size(s)=w1359:i32)
            n540 = Index Array(array=w1324, index=0) -> (element=w1321:i32)
            n541 = Index Array(array=w1324, index=1) -> (element=w1320:i32)
            n542 = for {
              N: w1359 -> [_]
              tunnel: w1325 -> [w1368] mode=indexing
              tunnel: [w1366] -> w1348 mode=indexing
              # "This loop add a F for each Y moviment"
              n543 = Build Array (concatenate)(w1368, FALSE) -> (w1366:bool[])
            }
            "Laser on/off array" <- w1348
            n544 = Multiply(x=w1321, y=w1320) -> (x*y=w1319:i32)
            n545 = Multiply(x=w1319, y=w1318) -> (x*y=w1317:dbl)
            n546 = Round To Nearest(number=w1311) -> (nearest integer value=w1309:dbl)
            n547 = local read "Speed (µm/s)"() -> (w1326:i32)
            n548 = local read "Axis 1"() -> (w1328:string)
            n549 = local read "Axis 2"() -> (w1327:string)
            n550 = call "Commands array generator.vi"("Axis 1"=w1328, "Axis in"=w1327, "Axes speed \n(µm/s)"=w1326, "Y Step size in µm"=w1309, "T/F product array"=w1325, "Space defined array"=w1298) -> ("Command Array"=→"Commands array":string[][], "Time Array"=w1329:dbl[][])  [unwired: 4 in]
            n551 = Add Array Elements(numeric array=w1329) -> (sum=w1316:dbl)
            n552 = Add(x=w1317, y=w1316) -> (x+y=w1315:dbl)
            "Processi time (sec)" <- w1315
            n553 = local write "Process time"(w1315) -> ()
          }
        }
      }
      event "Call Last ROI": Value Change {
        n554 = event-data() -> ()  [unwired: 1 in, 6 out]
        n555 = control-ref of="This VI"() -> (w1376:refnum<vi>)
        n556 = property class="VI"(reference=w1376) -> ("Path"=w1373:path)  [unwired: 1 in, 2 out]
        n557 = Strip Path(path=w1373) -> (stripped path=w1374:path)  [unwired: 1 out]
        n558 = Build Path(base path=w1374, name or relative path="Last_ROI.TIFF") -> (appended path=w1370:path)
        n559 = call <vilib>:"Check if File or Folder Exists.vi"("path"=w1370) -> ("file or folder exists?"=w1371:bool)  [unwired: 8 in, 2 out]
        n560 = And(x=w1371, y="Call Last ROI") -> (x .and. y?=w1369:bool)
        n561 = case shown="True" w1369 {
          tunnel: w1370 -> [_ w1384]
          frame False {
          }
          frame True {
            n562 = call "IMAQ Create"("Image Name"="untitled") -> ("New Image"=w1386:T2)  [unwired: 4 in, 1 out]
            n563 = call "IMAQ ReadFile"("File Path"=w1384, "Image"=w1386) -> ("Image Out"=w1385:T2)  [unwired: 5 in, 4 out]
            n564 = call "IMAQ MaskToROI"("Image"=w1385) -> ("ROI Descriptor"=w1377:T13)  [unwired: 6 in, 2 out]
            n565 = Unbundle By Name(w1377) -> ("Contours"=w1382:T14)  [unwired: 1 out]
            n566 = Index Array(array=w1382) -> (element=w1383:T15)  [unwired: 1 in]
            n567 = Bundle By Name(cluster=w1383, "Type"=u32 6) -> (w1381:T15)
            n568 = Replace Array Subset(array=w1382, new element=w1381) -> (w1380:T14)  [unwired: 1 in]
            n569 = Bundle By Name(cluster=w1377, "Contours"=w1380) -> (w1378:T13)
            n570 = property on="Source" class="ImageControl"("ROI"=w1378) -> ()  [unwired: 2 in, 2 out]
          }
        }
      }
      event "Save current ROI": Value Change {
        n571 = event-data() -> ()  [unwired: 1 in, 6 out]
        n572 = property on="Source" class="ImageControl"() -> ("ROI"=w1389:T11)  [unwired: 2 in, 2 out]
        n573 = Unbundle By Name(w1389) -> ("Contours"=w1394:T16)
        n574 = Index Array(array=w1394) -> (element=w1393:T17)  [unwired: 1 in]
        n575 = Unbundle By Name(w1393) -> ("ROI Type"=w1392:u32)
        n576 = Not Equal To 0?(x=w1392) -> (x != 0?=w1391:bool)
        n577 = And(x="Save current ROI", y=w1391) -> (x .and. y?=w1388:bool)
        n578 = case shown="True" w1388 {
          tunnel: w1389 -> [_ w1405]
          frame False {
          }
          frame True {
            n579 = control-ref of="This VI"() -> (w1409:refnum<vi>)
            n580 = property class="VI"(reference=w1409) -> ("Path"=w1410:path)  [unwired: 1 in, 2 out]
            n581 = call "IMAQ Create"("Image Name"="untitled") -> ("New Image"=w1406:T2)  [unwired: 4 in, 1 out]
            n582 = call "IMAQ ROIToMask 2"("ROI Descriptor"=w1405, "Image"=w1406) -> ("Image Out"=w1408:T2)  [unwired: 7 in, 2 out]
            n583 = Strip Path(path=w1410) -> (stripped path=w1411:path)  [unwired: 1 out]
            n584 = Build Path(base path=w1411, name or relative path="Saved ROI") -> (appended path=w1404:path)